vi "Dresden R2R Sputter 03.02.2018 IY24.vi"() -> ()   [LabVIEW 2009] (continued)
          }
          frame #9 {
            n6832 = flat-sequence {
              frame #0 {
                n6833 = Wait (ms)(milliseconds to wait=i32? 100) -> ()  [unwired: 1 out]
              }
              frame #1 {
                n6834 = local write "DC_auto_voltage_mode"(i16? 0 ("DC_auto_voltage_mode")) -> ()
              }
            }
            n6835 = VISA Write(VISA resource name=w10558, write buffer=bytes[4], error in (no error)=w10557) -> (VISA resource name out=w10556, error out=w10555)  [unwired: 1 out]
          }
        }
      }
    }
  }
  n6836 = call <vilib>:"MB Serial Init.vi"("Timeout"=i32? 2000, "Mode"=w750, "Parity"=w752, "Baud Rate"=i32? 9600, "VISA resource name"="Moxa I/O Ch 4") -> ("error out"=w756:errorcluster, "VISA resource name out"=w755:refnum<visa-resource-name>)  [unwired: 2 in, 3 out]
  n6837 = call <vilib>:"MB Serial Init.vi"("Timeout"=i32? 2000, "Mode"=w766, "Parity"=w764, "Baud Rate"=i32? 9600, "VISA resource name"="Moxa I/O Ch 3") -> ("error out"=w760:errorcluster, "VISA resource name out"=w761:refnum<visa-resource-name>)  [unwired: 2 in, 3 out]
  n6838 = while {
    tunnel: w814 -> [w10986]
    tunnel: w813 -> [w10985]
    shift-right: [w10811] -> _
    shift-left: _ -> [w10810]
    tunnel: [w10734] -> w809
    tunnel: [w10733] -> w733
    stop <- i16? 0 stop-if-true
    w10624 = bytes[2]
    w10586 = bytes[2]
    # "guc kaynagı ACK gelınceye kadar bekler."
    # "ACK karsılıgı 06(hex) dır."
    n6839 = Tick Count (ms)() -> (millisecond timer value=w10811)
    n6840 = Or(x="set rf", y="RF set auto") -> (x .or. y?=w10570)
    n6841 = Or(x="RF on", y="RF_auto_on") -> (x .or. y?=w10581)
    n6842 = Or(x="oto tuner", y="RF_auto_tuner") -> (x .or. y?=w10562)
    n6843 = Or(x="RF off", y="RF_auto_off") -> (x .or. y?=w10579)
    n6844 = Or(x="RF host", y="RF_host_auto") -> (x .or. y?=w10576)
    n6845 = Subtract(x=w10811, y=w10810) -> (x-y=→"x-y")
    n6846 = Or(x="Ramp Up time", y="Ramp Up time_auto") -> (x .or. y?=w10574)
    n6847 = Boolean To (0,1)(Boolean=w10576) -> (0, 1=w10960)
    n6848 = Boolean To (0,1)(Boolean=w10579) -> (0, 1=w10961)
    n6849 = Boolean To (0,1)(Boolean=w10581) -> (0, 1=w10967)
    n6850 = Boolean To (0,1)(Boolean=w10570) -> (0, 1=w10966)
    n6851 = Boolean To (0,1)(Boolean=w10562) -> (0, 1=w10965)
    n6852 = Boolean To (0,1)(Boolean="initialize") -> (0, 1=w10963)
    n6853 = Boolean To (0,1)(Boolean="Load") -> (0, 1=w10688)
    n6854 = Boolean To (0,1)(Boolean="Forward") -> (0, 1=w10685)
    n6855 = Boolean To (0,1)(Boolean="External") -> (0, 1=w10691)
    n6856 = Boolean To (0,1)(Boolean="Pulsing_off") -> (0, 1=w10698)
    n6857 = Boolean To (0,1)(Boolean="internal") -> (0, 1=w10699)
    n6858 = Boolean To (0,1)(Boolean="external") -> (0, 1=w10701)
    n6859 = Boolean To (0,1)(Boolean="set duty") -> (0, 1=w10714)
    n6860 = Boolean To (0,1)(Boolean=w10574) -> (0, 1=w10673)
    n6861 = Boolean To (0,1)(Boolean="manuel tuner") -> (0, 1=w10964)
    n6862 = Boolean To (0,1)(Boolean="set cap pos") -> (0, 1=w10962)
    n6863 = Boolean To (0,1)(Boolean="set seri cap pos 2") -> (0, 1=w10959)
    n6864 = Boolean To (0,1)(Boolean="set frequency") -> (0, 1=w10710)
    n6865 = Multiply(x=w10960, y=i16? 1) -> (x*y=w10683)
    n6866 = Multiply(x=w10961, y=i16? 3) -> (x*y=w10980)
    n6867 = Multiply(x=w10967, y=i16? 4) -> (x*y=w10981)
    n6868 = Multiply(x=w10966, y=i16? 5) -> (x*y=w10978)
    n6869 = Multiply(x=w10965, y=i16? 6) -> (x*y=w10976)
    n6870 = Multiply(x=w10963, y=i16? 8) -> (x*y=w10972)
    n6871 = Or(x="Ramp down time", y="Ramp Down time_auto") -> (x .or. y?=w10569)
    n6872 = Boolean To (0,1)(Boolean=w10569) -> (0, 1=w10671)
    n6873 = Multiply(x=w10964, y=i16? 7) -> (x*y=w10974)
    n6874 = Multiply(x=w10962, y=i16? 9) -> (x*y=w10970)
    n6875 = Multiply(x=w10688, y=i16? 2) -> (x*y=w10708)
    n6876 = Multiply(x=w10959, y=i16? 10) -> (x*y=w10968)
    n6877 = Multiply(x=w10685, y=i16? 11) -> (x*y=w10707)
    n6878 = Multiply(x=w10691, y=i16? 12) -> (x*y=w10706)
    n6879 = Multiply(x=w10698, y=i16? 13) -> (x*y=w10703)
    n6880 = Multiply(x=w10699, y=i16? 14) -> (x*y=w10704)
    n6881 = Multiply(x=w10701, y=i16? 15) -> (x*y=w10705)
    n6882 = Multiply(x=w10710, y=i16? 16) -> (x*y=w10712)
    n6883 = Multiply(x=w10714, y=i16? 17) -> (x*y=w10716)
    n6884 = Multiply(x=w10673, y=i16? 18) -> (x*y=w10670)
    n6885 = Multiply(x=w10671, y=i16? 19) -> (x*y=w10669)
    n6886 = String To Byte Array(string=w10586) -> (unsigned byte array=w10668)
    n6887 = for {
      tunnel: w10668 -> [w11022] mode=indexing
      shift-right: [w11020] -> w10666
      shift-left: data[5B] -> [w11021]
      n6888 = Exclusive Or(1:w11021, 2:w11022) -> (0:w11020)
    }
    n6889 = Compound Arithmetic op=ADD(w10708, w10707, w10706, w10703, w10704, w10705, w10712, w10716) -> (w10684)
    n6890 = Build Array(w10666) -> (w10665)
    n6891 = Compound Arithmetic op=ADD(w10683, w10980, w10981, w10978, w10976, w10974, w10972, w10970, w10968, w10684, w10670, w10669) -> (w10956)
    n6892 = Byte Array To String(unsigned byte array=w10665) -> (string=w10664)
    n6893 = Not Equal To 0?(x=w10956) -> (x != 0?=w10955)
    n6894 = case shown="3" w10956 {
      tunnel: [w11133 w11138 w11141 w11155 w11161 w11168 w11192 w11207 w11223 w11243 w11268 w11284 w11298 w11312 w11326 w11340 w11354 w11382 w11402 w11427] -> w10958
      tunnel: [w11132 w11137 w11140 w11156 w11162 w11169 w11191 w11206 w11224 w11242 w11267 w11283 w11297 w11311 w11325 w11339 w11353 w11381 w11401 w11426] -> w10957
      tunnel: w10986 -> [w11133 w11136 w11143 w11158 w11164 w11171 w11194 w11209 w11222 w11245 w11270 w11286 w11300 w11314 w11328 w11342 w11356 w11384 w11404 w11429]
      tunnel: w10985 -> [w11132 w11135 w11142 w11157 w11163 w11170 w11193 w11208 w11221 w11244 w11269 w11285 w11299 w11313 w11327 w11341 w11355 w11383 w11403 w11428]
      frame #0 {
      }
      frame #1 {
        # "Host kontrol"
        n6895 = local write "RF_host_auto"(i16? 0 ("RF_host_auto")) -> ()
        n6896 = VISA Write(VISA resource name=w11136, write buffer=bytes[4], error in (no error)=w11135) -> (VISA resource name out=w11138, error out=w11137)  [unwired: 1 out]
      }
      frame #2 {
        w11150 = bytes[3]
        n6897 = String To Byte Array(string=w11150) -> (unsigned byte array=w11144)
        n6898 = for {
          tunnel: w11144 -> [w11153] mode=indexing
          shift-right: [w11151] -> w11146
          shift-left: data[5B] -> [w11152]
          n6899 = Exclusive Or(1:w11152, 2:w11153) -> (0:w11151)
        }
        n6900 = Build Array(w11146) -> (w11148)
        n6901 = Byte Array To String(unsigned byte array=w11148) -> (string=w11147)
        n6902 = Concatenate Strings(w11150, w11147) -> (w11149)
        n6903 = VISA Write(VISA resource name=w11143, write buffer=w11149, error in (no error)=w11142) -> (VISA resource name out=w11141, error out=w11140)  [unwired: 1 out]
      }
      frame #3 {
        # "RF OFF"
        n6904 = local write "RF_auto_off"(i16? 0 ("RF_auto_off")) -> ()
        n6905 = VISA Write(VISA resource name=w11158, write buffer=bytes[3], error in (no error)=w11157) -> (VISA resource name out=w11155, error out=w11156)  [unwired: 1 out]
      }
      frame #4 {
        # "RF ON"
        n6906 = local write "RF_auto_on"(i16? 0 ("RF_auto_on")) -> ()
        n6907 = VISA Write(VISA resource name=w11164, write buffer=bytes[3], error in (no error)=w11163) -> (VISA resource name out=w11161, error out=w11162)  [unwired: 1 out]
      }
      frame #5 {
        n6908 = local write "RF set auto"(i16? 0 ("RF set auto")) -> ()
        n6909 = Quotient & Remainder(x="RF_forward_power_1", y=dbl? 256.0) -> (x-y*floor(x/y)=w11178, floor(x/y)=w11174)
        n6910 = Build Array(w11178) -> (w11177)
        n6911 = Build Array(w11174) -> (w11175)
        n6912 = Byte Array To String(unsigned byte array=w11177) -> (string=w11176)
        n6913 = Byte Array To String(unsigned byte array=w11175) -> (string=w11173)
        n6914 = Concatenate Strings(bytes[2], w11176, w11173) -> (w11180)
        n6915 = String To Byte Array(string=w11180) -> (unsigned byte array=w11186)
        n6916 = for {
          tunnel: w11186 -> [w11189] mode=indexing
          shift-right: [w11187] -> w11184
          shift-left: data[5B] -> [w11188]
          n6917 = Exclusive Or(1:w11188, 2:w11189) -> (0:w11187)
        }
        n6918 = Build Array(w11184) -> (w11183)
        n6919 = Byte Array To String(unsigned byte array=w11183) -> (string=w11181)
        n6920 = Concatenate Strings(w11180, w11181) -> (w11172)
        n6921 = VISA Write(VISA resource name=w11171, write buffer=w11172, error in (no error)=w11170) -> (VISA resource name out=w11168, error out=w11169)  [unwired: 1 out]
      }
      frame #6 {
        n6922 = Concatenate Strings(bytes[3]) -> (w11196)
        n6923 = local write "RF_auto_tuner"(i16? 0 ("RF_auto_tuner")) -> ()
        n6924 = String To Byte Array(string=w11196) -> (unsigned byte array=w11202)
        n6925 = for {
          tunnel: w11202 -> [w11205] mode=indexing
          shift-right: [w11203] -> w11200
          shift-left: data[5B] -> [w11204]
          n6926 = Exclusive Or(1:w11204, 2:w11205) -> (0:w11203)
        }
        n6927 = Build Array(w11200) -> (w11199)
        n6928 = Byte Array To String(unsigned byte array=w11199) -> (string=w11197)
        n6929 = Concatenate Strings(w11196, w11197) -> (w11195)
        n6930 = VISA Write(VISA resource name=w11194, write buffer=w11195, error in (no error)=w11193) -> (VISA resource name out=w11192, error out=w11191)  [unwired: 1 out]
      }
      frame #7 {
        n6931 = Concatenate Strings(bytes[3]) -> (w11211)
        n6932 = String To Byte Array(string=w11211) -> (unsigned byte array=w11217)
        n6933 = for {
          tunnel: w11217 -> [w11220] mode=indexing
          shift-right: [w11218] -> w11215
          shift-left: data[5B] -> [w11219]
          n6934 = Exclusive Or(1:w11219, 2:w11220) -> (0:w11218)
        }
        n6935 = Build Array(w11215) -> (w11214)
        n6936 = Byte Array To String(unsigned byte array=w11214) -> (string=w11212)
        n6937 = Concatenate Strings(w11211, w11212) -> (w11210)
        n6938 = VISA Write(VISA resource name=w11209, write buffer=w11210, error in (no error)=w11208) -> (VISA resource name out=w11207, error out=w11206)  [unwired: 1 out]
      }
      frame #8 {
        w11228 = bytes[2]
        n6939 = String To Byte Array(string=w11228) -> (unsigned byte array=w11231)
        n6940 = for {
          tunnel: w11231 -> [w11234] mode=indexing
          shift-right: [w11232] -> w11229
          shift-left: data[5B] -> [w11233]
          n6941 = Exclusive Or(1:w11233, 2:w11234) -> (0:w11232)
        }
        n6942 = Build Array(w11229) -> (w11226)
        n6943 = Byte Array To String(unsigned byte array=w11226) -> (string=w11227)
        n6944 = Concatenate Strings(w11228, w11227) -> (w11225)
        n6945 = VISA Write(VISA resource name=w11222, write buffer=w11225, error in (no error)=w11221) -> (VISA resource name out=w11223, error out=w11224)  [unwired: 1 out]
      }
      frame #9 {
        n6946 = Multiply(x="Set CL Position:", y=dbl? 10.0) -> (x*y=w11237)
        n6947 = To Unsigned Long Integer(number=w11237) -> (unsigned 32bit integer=w11236)
        n6948 = Quotient & Remainder(x=w11236, y=i32? 256) -> (x-y*floor(x/y)=w11241, floor(x/y)=w11240)
        n6949 = Build Array(w11241, w11240) -> (w11248)
        n6950 = Byte Array To String(unsigned byte array=w11248) -> (string=w11247)
        n6951 = Concatenate Strings("\np", w11247) -> (w11249)
        n6952 = String To Byte Array(string=w11249) -> (unsigned byte array=w11255)
        n6953 = for {
          tunnel: w11255 -> [w11258] mode=indexing
          shift-right: [w11256] -> w11253
          shift-left: data[5B] -> [w11257]
          n6954 = Exclusive Or(1:w11257, 2:w11258) -> (0:w11256)
        }
        n6955 = Build Array(w11253) -> (w11252)
        n6956 = Byte Array To String(unsigned byte array=w11252) -> (string=w11250)
        n6957 = Concatenate Strings(w11249, w11250) -> (w11246)
        n6958 = VISA Write(VISA resource name=w11245, write buffer=w11246, error in (no error)=w11244) -> (VISA resource name out=w11243, error out=w11242)  [unwired: 1 out]
      }
      frame #10 {
        n6959 = Multiply(x="Set CT Position:", y=dbl? 10.0) -> (x*y=w11259)
        n6960 = To Unsigned Long Integer(number=w11259) -> (unsigned 32bit integer=w11260)
        n6961 = Quotient & Remainder(x=w11260, y=i32? 256) -> (x-y*floor(x/y)=w11265, floor(x/y)=w11264)
        n6962 = Build Array(w11265, w11264) -> (w11262)
        n6963 = Byte Array To String(unsigned byte array=w11262) -> (string=w11272)
        n6964 = Concatenate Strings("\nz", w11272) -> (w11273)
        n6965 = String To Byte Array(string=w11273) -> (unsigned byte array=w11279)
        n6966 = for {
          tunnel: w11279 -> [w11282] mode=indexing
          shift-right: [w11280] -> w11277
          shift-left: data[5B] -> [w11281]
          n6967 = Exclusive Or(1:w11281, 2:w11282) -> (0:w11280)
        }
        n6968 = Build Array(w11277) -> (w11276)
        n6969 = Byte Array To String(unsigned byte array=w11276) -> (string=w11274)
        n6970 = Concatenate Strings(w11273, w11274) -> (w11271)
        n6971 = VISA Write(VISA resource name=w11270, write buffer=w11271, error in (no error)=w11269) -> (VISA resource name out=w11268, error out=w11267)  [unwired: 1 out]
      }
      frame #11 {
        w11290 = bytes[3]
        n6972 = String To Byte Array(string=w11290) -> (unsigned byte array=w11287)
        n6973 = for {
          tunnel: w11287 -> [w11296] mode=indexing
          shift-right: [w11294] -> w11289
          shift-left: data[5B] -> [w11295]
          n6974 = Exclusive Or(1:w11295, 2:w11296) -> (0:w11294)
        }
        n6975 = Build Array(w11289) -> (w11291)
        n6976 = Byte Array To String(unsigned byte array=w11291) -> (string=w11292)
        n6977 = Concatenate Strings(w11290, w11292) -> (w11293)
        n6978 = VISA Write(VISA resource name=w11286, write buffer=w11293, error in (no error)=w11285) -> (VISA resource name out=w11284, error out=w11283)  [unwired: 1 out]
      }
      frame #12 {
        w11305 = bytes[3]
        n6979 = String To Byte Array(string=w11305) -> (unsigned byte array=w11301)
        n6980 = for {
          tunnel: w11301 -> [w11310] mode=indexing
          shift-right: [w11308] -> w11303
          shift-left: data[5B] -> [w11309]
          n6981 = Exclusive Or(1:w11309, 2:w11310) -> (0:w11308)
        }
        n6982 = Build Array(w11303) -> (w11304)
        n6983 = Byte Array To String(unsigned byte array=w11304) -> (string=w11306)
        n6984 = Concatenate Strings(w11305, w11306) -> (w11307)
        n6985 = VISA Write(VISA resource name=w11300, write buffer=w11307, error in (no error)=w11299) -> (VISA resource name out=w11298, error out=w11297)  [unwired: 1 out]
      }
      frame #13 {
        w11319 = bytes[3]
        n6986 = String To Byte Array(string=w11319) -> (unsigned byte array=w11315)
        n6987 = for {
          tunnel: w11315 -> [w11324] mode=indexing
          shift-right: [w11322] -> w11317
          shift-left: data[5B] -> [w11323]
          n6988 = Exclusive Or(1:w11323, 2:w11324) -> (0:w11322)
        }
        n6989 = Build Array(w11317) -> (w11318)
        n6990 = Byte Array To String(unsigned byte array=w11318) -> (string=w11320)
        n6991 = Concatenate Strings(w11319, w11320) -> (w11321)
        n6992 = VISA Write(VISA resource name=w11314, write buffer=w11321, error in (no error)=w11313) -> (VISA resource name out=w11312, error out=w11311)  [unwired: 1 out]
      }
      frame #14 {
        w11335 = bytes[3]
        n6993 = String To Byte Array(string=w11335) -> (unsigned byte array=w11329)
        n6994 = for {
          tunnel: w11329 -> [w11338] mode=indexing
          shift-right: [w11336] -> w11331
          shift-left: data[5B] -> [w11337]
          n6995 = Exclusive Or(1:w11337, 2:w11338) -> (0:w11336)
        }
        n6996 = Build Array(w11331) -> (w11332)
        n6997 = Byte Array To String(unsigned byte array=w11332) -> (string=w11333)
        n6998 = Concatenate Strings(w11335, w11333) -> (w11334)
        n6999 = VISA Write(VISA resource name=w11328, write buffer=w11334, error in (no error)=w11327) -> (VISA resource name out=w11326, error out=w11325)  [unwired: 1 out]
      }
      frame #15 {
        w11347 = bytes[3]
        n7000 = String To Byte Array(string=w11347) -> (unsigned byte array=w11343)
        n7001 = for {
          tunnel: w11343 -> [w11352] mode=indexing
          shift-right: [w11350] -> w11345
          shift-left: data[5B] -> [w11351]
          n7002 = Exclusive Or(1:w11351, 2:w11352) -> (0:w11350)
        }
        n7003 = Build Array(w11345) -> (w11346)
        n7004 = Byte Array To String(unsigned byte array=w11346) -> (string=w11348)
        n7005 = Concatenate Strings(w11347, w11348) -> (w11349)
        n7006 = VISA Write(VISA resource name=w11342, write buffer=w11349, error in (no error)=w11341) -> (VISA resource name out=w11340, error out=w11339)  [unwired: 1 out]
      }
      frame #16 {
        w11369 = dbl? 256.0 ("y")
        n7007 = Quotient & Remainder(x="Frequency :", y=w11369) -> (x-y*floor(x/y)=w11364, floor(x/y)=w11368)
        n7008 = Build Array(w11364) -> (w11365)
        n7009 = Quotient & Remainder(x=w11368, y=w11369) -> (x-y*floor(x/y)=w11370, floor(x/y)=w11374)
        n7010 = Byte Array To String(unsigned byte array=w11365) -> (string=w11372)
        n7011 = Build Array(w11370) -> (w11371)
        n7012 = Build Array(w11374) -> (w11366)
        n7013 = Byte Array To String(unsigned byte array=w11371) -> (string=w11375)
        n7014 = Byte Array To String(unsigned byte array=w11366) -> (string=w11376)
        n7015 = Concatenate Strings(bytes[2], w11372, w11375, w11376, bytes[1] ("string")) -> (w11363)
        n7016 = String To Byte Array(string=w11363) -> (unsigned byte array=w11357)
        n7017 = for {
          tunnel: w11357 -> [w11380] mode=indexing
          shift-right: [w11378] -> w11359
          shift-left: data[5B] -> [w11379]
          n7018 = Exclusive Or(1:w11379, 2:w11380) -> (0:w11378)
        }
        n7019 = Build Array(w11359) -> (w11360)
        n7020 = Byte Array To String(unsigned byte array=w11360) -> (string=w11362)
        n7021 = Concatenate Strings(w11363, w11362) -> (w11377)
        n7022 = VISA Write(VISA resource name=w11356, write buffer=w11377, error in (no error)=w11355) -> (VISA resource name out=w11354, error out=w11353)  [unwired: 1 out]
      }
      frame #17 {
        n7023 = Build Array("Duty Cycle :") -> (w11394)
        n7024 = Byte Array To String(unsigned byte array=w11394) -> (string=w11395)
        n7025 = Concatenate Strings("\n`", w11395, bytes[1] ("string")) -> (w11391)
        n7026 = String To Byte Array(string=w11391) -> (unsigned byte array=w11385)
        n7027 = for {
          tunnel: w11385 -> [w11399] mode=indexing
          shift-right: [w11397] -> w11387
          shift-left: data[5B] -> [w11398]
          n7028 = Exclusive Or(1:w11398, 2:w11399) -> (0:w11397)
        }
        n7029 = Build Array(w11387) -> (w11388)
        n7030 = Byte Array To String(unsigned byte array=w11388) -> (string=w11390)
        n7031 = Concatenate Strings(w11391, w11390) -> (w11396)
        n7032 = VISA Write(VISA resource name=w11384, write buffer=w11396, error in (no error)=w11383) -> (VISA resource name out=w11382, error out=w11381)  [unwired: 1 out]
      }
      frame #18 {
        n7033 = Multiply(x="Ramp up Time:", y=dbl? 10.0) -> (x*y=w11408)
        n7034 = To Unsigned Long Integer(number=w11408) -> (unsigned 32bit integer=w11407)
        n7035 = local write "Ramp Up time_auto"(i16? 0 ("Ramp Up time_auto")) -> ()
        n7036 = Quotient & Remainder(x=w11407, y=i32? 256) -> (x-y*floor(x/y)=w11411, floor(x/y)=w11410)
        n7037 = Build Array(w11411, w11410) -> (w11406)
        n7038 = Byte Array To String(unsigned byte array=w11406) -> (string=w11414)
        n7039 = Concatenate Strings(bytes[2], w11414) -> (w11415)
        n7040 = String To Byte Array(string=w11415) -> (unsigned byte array=w11421)
        n7041 = for {
          tunnel: w11421 -> [w11424] mode=indexing
          shift-right: [w11422] -> w11419
          shift-left: data[5B] -> [w11423]
          n7042 = Exclusive Or(1:w11423, 2:w11424) -> (0:w11422)
        }
        n7043 = Build Array(w11419) -> (w11418)
        n7044 = Byte Array To String(unsigned byte array=w11418) -> (string=w11416)
        n7045 = Concatenate Strings(w11415, w11416) -> (w11413)
        n7046 = VISA Write(VISA resource name=w11404, write buffer=w11413, error in (no error)=w11403) -> (VISA resource name out=w11402, error out=w11401)  [unwired: 1 out]
      }
      frame #19 {
        n7047 = Multiply(x="Ramp Down Time :", y=dbl? 10.0) -> (x*y=w11433)
        n7048 = To Unsigned Long Integer(number=w11433) -> (unsigned 32bit integer=w11432)
        n7049 = local write "Ramp Down time_auto"(i16? 0 ("Ramp Down time_auto")) -> ()
        n7050 = Quotient & Remainder(x=w11432, y=i32? 256) -> (x-y*floor(x/y)=w11436, floor(x/y)=w11435)
        n7051 = Build Array(w11436, w11435) -> (w11431)
        n7052 = Byte Array To String(unsigned byte array=w11431) -> (string=w11439)
        n7053 = Concatenate Strings("\n ", w11439) -> (w11440)
        n7054 = String To Byte Array(string=w11440) -> (unsigned byte array=w11446)
        n7055 = for {
          tunnel: w11446 -> [w11449] mode=indexing
          shift-right: [w11447] -> w11444
          shift-left: data[5B] -> [w11448]
          n7056 = Exclusive Or(1:w11448, 2:w11449) -> (0:w11447)
        }
        n7057 = Build Array(w11444) -> (w11443)
        n7058 = Byte Array To String(unsigned byte array=w11443) -> (string=w11441)
        n7059 = Concatenate Strings(w11440, w11441) -> (w11438)
        n7060 = VISA Write(VISA resource name=w11429, write buffer=w11438, error in (no error)=w11428) -> (VISA resource name out=w11427, error out=w11426)  [unwired: 1 out]
      }
    }
    n7061 = Concatenate Strings(w10586, w10664) -> (w10657)
    n7062 = case shown="True" w10955 {
      tunnel: w10958 -> [w11116 w11126]
      tunnel: w10957 -> [w11115 w11125]
      tunnel: [w11116 w11128] -> w10945
      tunnel: [w11115 w11122] -> w10944
      frame #0 {
      }
      frame #1 {
        n7063 = stacked-sequence {
          tunnel: [w11131] -> w11124
          tunnel: w11126 -> [w11131]
          tunnel: [w11130] -> w11123
          tunnel: w11125 -> [w11130]
          frame #0 {
            n7064 = Wait Until Next ms Multiple(millisecond multiple=i32? 40) -> ()  [unwired: 1 out]
          }
        }
        n7065 = property class="Instr"(reference=w11124, error in=w11123) -> (reference out=w11121, error out=w11120, "Serial Settings:Number of Bytes at Serial Port"=w11119)
        n7066 = VISA Read(VISA resource name=w11121, byte count=w11119, error in (no error)=w11120) -> (VISA resource name out=w11118, error out=w11117)  [unwired: 2 out]
        n7067 = VISA Write(VISA resource name=w11118, write buffer=bytes[1], error in (no error)=w11117) -> (VISA resource name out=w11128, error out=w11122)  [unwired: 1 out]
      }
    }
    n7068 = VISA Write(VISA resource name=w10945, write buffer=bytes[3], error in (no error)=w10944) -> (VISA resource name out=w10950, error out=w10949)  [unwired: 1 out]
    n7069 = stacked-sequence {
      tunnel: [w11114] -> w10947
      tunnel: w10950 -> [w11114]
      tunnel: [w11113] -> w10946
      tunnel: w10949 -> [w11113]
      frame #0 {
        n7070 = Wait Until Next ms Multiple(millisecond multiple=i32? 40) -> ()  [unwired: 1 out]
      }
    }
    n7071 = property class="Instr"(reference=w10947, error in=w10946) -> (reference out=w10951, error out=w10953, "Serial Settings:Number of Bytes at Serial Port"=w10952)
    n7072 = VISA Read(VISA resource name=w10951, byte count=w10952, error in (no error)=w10953) -> (VISA resource name out=w10595, read buffer=w10943, error out=w10594)  [unwired: 1 out]
    n7073 = Match Pattern(string=w10943, regular expression="¦") -> (after substring=w10591)  [unwired: 4 out]
    n7074 = String Length(string=w10591) -> (length=w10942)
    n7075 = String Subset(string=w10591, length (rest)=i32? 2 ("length (rest)")) -> (substring=w10940)  [unwired: 1 out]
    n7076 = Not Equal To 0?(x=w10942) -> (x != 0?=w10588)
    n7077 = String To Byte Array(string=w10940) -> (unsigned byte array=w10938)
    n7078 = case shown="True" w10588 {
      tunnel: [w10989 w10993] -> w10593
      tunnel: [w10988 w10992] -> w10592
      tunnel: w10595 -> [w10989 w10991]
      tunnel: w10594 -> [w10988 w10990]
      frame #0 {
      }
      frame #1 {
        n7079 = VISA Write(VISA resource name=w10991, write buffer=bytes[1], error in (no error)=w10990) -> (VISA resource name out=w10993, error out=w10992)  [unwired: 1 out]
      }
    }
    n7080 = Index Array(array=w10938, index=i32? 1) -> (element=w10934)
    n7081 = Index Array(array=w10938, index=data[5B]) -> (element=w10932)
    n7082 = To Unsigned Long Integer(number=w10934) -> (unsigned 32bit integer=w10936)
    n7083 = To Unsigned Long Integer(number=w10932) -> (unsigned 32bit integer=w10931)
    n7084 = Multiply(x=i32? 256, y=w10936) -> (x*y=w10933)
    n7085 = Add(x=w10933, y=w10931) -> (x+y=w10682)
    n7086 = case shown="True" w10588 {
      tunnel: w10682 -> [_ w11041]
      frame #0 {
      }
      frame #1 {
        "Reflected Power" <- w11041
      }
    }
    n7087 = VISA Write(VISA resource name=w10593, write buffer=w10657, error in (no error)=w10592) -> (VISA resource name out=w10661, error out=w10660)  [unwired: 1 out]
    n7088 = stacked-sequence {
      tunnel: [w11019] -> w10659
      tunnel: w10661 -> [w11019]
      tunnel: [w11018] -> w10658
      tunnel: w10660 -> [w11018]
      frame #0 {
        n7089 = Wait Until Next ms Multiple(millisecond multiple=i32? 40) -> ()  [unwired: 1 out]
      }
    }
    n7090 = property class="Instr"(reference=w10659, error in=w10658) -> (reference out=w10662, error out=w10663, "Serial Settings:Number of Bytes at Serial Port"=w10587)
    n7091 = VISA Read(VISA resource name=w10662, byte count=w10587, error in (no error)=w10663) -> (VISA resource name out=w10644, read buffer=w10654, error out=w10643)  [unwired: 1 out]
    n7092 = Match Pattern(string=w10654, regular expression="¢") -> (after substring=w10652)  [unwired: 4 out]
    n7093 = String Length(string=w10652) -> (length=w10656)
    n7094 = String Subset(string=w10652, length (rest)=i32? 1 ("length (rest)")) -> (substring=w10650)  [unwired: 1 out]
    n7095 = String To Byte Array(string=w10650) -> (unsigned byte array=w10649)
    n7096 = Not Equal To 0?(x=w10656) -> (x != 0?=w10655)
    n7097 = Index Array(array=w10649, index=data[5B]) -> (element=w10647)
    n7098 = String To Byte Array(string=w10624) -> (unsigned byte array=w10629)
    n7099 = Number To Boolean Array(number=w10647) -> (Boolean array=w10646)
    n7100 = case shown="True" w10655 {
      tunnel: [w11011 w11015] -> w10597
      tunnel: [w11010 w11014] -> w10596
      tunnel: w10644 -> [w11011 w11013]
      tunnel: w10643 -> [w11010 w11012]
      frame #0 {
      }
      frame #1 {
        n7101 = VISA Write(VISA resource name=w11013, write buffer=bytes[1], error in (no error)=w11012) -> (VISA resource name out=w11015, error out=w11014)  [unwired: 1 out]
      }
    }
    n7102 = for {
      tunnel: w10629 -> [w10999] mode=indexing
      shift-right: [w10997] -> w10627
      shift-left: data[5B] -> [w10998]
      n7103 = Exclusive Or(1:w10998, 2:w10999) -> (0:w10997)
    }
    n7104 = Index Array(array=w10646, index=i32? 6) -> (element=→"RF 1 On")
    n7105 = Build Array(w10627) -> (w10626)
    n7106 = Byte Array To String(unsigned byte array=w10626) -> (string=w10625)
    n7107 = Concatenate Strings(w10624, w10625) -> (w10623)
    n7108 = VISA Write(VISA resource name=w10597, write buffer=w10623, error in (no error)=w10596) -> (VISA resource name out=w10639, error out=w10638)  [unwired: 1 out]
    n7109 = stacked-sequence {
      tunnel: [w11009] -> w10635
      tunnel: w10639 -> [w11009]
      tunnel: [w11008] -> w10634
      tunnel: w10638 -> [w11008]
      frame #0 {
        n7110 = Wait Until Next ms Multiple(millisecond multiple=i32? 40) -> ()  [unwired: 1 out]
      }
    }
    n7111 = property class="Instr"(reference=w10635, error in=w10634) -> (reference out=w10641, error out=w10640, "Serial Settings:Number of Bytes at Serial Port"=w10599)
    n7112 = VISA Read(VISA resource name=w10641, byte count=w10599, error in (no error)=w10640) -> (VISA resource name out=w10633, read buffer=w10636, error out=w10632)  [unwired: 1 out]
    n7113 = Match Pattern(string=w10636, regular expression="—") -> (after substring=w10630)  [unwired: 4 out]
    n7114 = String Length(string=w10630) -> (length=w10631)
    n7115 = String To Byte Array(string=w10630) -> (unsigned byte array=w10602)
    n7116 = Not Equal To 0?(x=w10631) -> (x != 0?=w10598)
    n7117 = Index Array(array=w10602, index=i32? 1) -> (element=w10618)
    n7118 = Index Array(array=w10602, index=data[5B]) -> (element=w10615)
    n7119 = Index Array(array=w10602, index=i32? 3) -> (element=w10613)
    n7120 = Index Array(array=w10602, index=i32? 2) -> (element=w10612)
    n7121 = To Unsigned Long Integer(number=w10618) -> (unsigned 32bit integer=w10617)
    n7122 = To Unsigned Long Integer(number=w10615) -> (unsigned 32bit integer=w10614)
    n7123 = To Unsigned Long Integer(number=w10613) -> (unsigned 32bit integer=w10610)
    n7124 = To Unsigned Long Integer(number=w10612) -> (unsigned 32bit integer=w10611)
    n7125 = case shown="True" w10598 {
      tunnel: w10633 -> [w11001 w11005]
      tunnel: w10632 -> [w11000 w11004]
      tunnel: [w11001 w11003] -> w10590
      tunnel: [w11000 w11002] -> w10589
      frame #0 {
      }
      frame #1 {
        n7126 = VISA Write(VISA resource name=w11005, write buffer=bytes[1], error in (no error)=w11004) -> (VISA resource name out=w11003, error out=w11002)  [unwired: 1 out]
      }
    }
    n7127 = local read "Forward Power"() -> (w10585)
    n7128 = local read "Reflected Power"() -> (w10584)
    n7129 = Multiply(x=w10617, y=i32? 256) -> (x*y=w10620)
    n7130 = Multiply(x=i32? 256, y=w10610) -> (x*y=w10608)
    n7131 = Add(x=w10620, y=w10614) -> (x+y=w10603)
    n7132 = Add(x=w10608, y=w10611) -> (x+y=w10604)
    n7133 = Subtract(x=w10585, y=w10584) -> (x-y=→"RF Net Power :")
    n7134 = Divide(x=w10603, y=i32? 10) -> (x/y=w10601)
    n7135 = Divide(x=w10604, y=i32? 10) -> (x/y=w10600)
    n7136 = case shown="True" w10598 {
      tunnel: w10601 -> [_ w10996]
      tunnel: w10600 -> [_ w10995]
      frame #0 {
      }
      frame #1 {
        "Ramp Up Left Time:" <- w10996
        "Ramp Down Left Time:" <- w10995
      }
    }
    n7137 = VISA Write(VISA resource name=w10590, write buffer=bytes[3], error in (no error)=w10589) -> (VISA resource name out=w10912, error out=w10910)  [unwired: 1 out]
    n7138 = stacked-sequence {
      tunnel: [w11110] -> w10913
      tunnel: w10912 -> [w11110]
      tunnel: [w11109] -> w10911
      tunnel: w10910 -> [w11109]
      frame #0 {
        n7139 = Wait Until Next ms Multiple(millisecond multiple=i32? 40) -> ()  [unwired: 1 out]
      }
    }
    n7140 = property class="Instr"(reference=w10913, error in=w10911) -> (reference out=w10928, error out=w10927, "Serial Settings:Number of Bytes at Serial Port"=w10929)
    n7141 = VISA Read(VISA resource name=w10928, byte count=w10929, error in (no error)=w10927) -> (VISA resource name out=w10909, read buffer=w10914, error out=w10908)  [unwired: 1 out]
    n7142 = Match Pattern(string=w10914, regular expression="¥") -> (after substring=w10906)  [unwired: 4 out]
    n7143 = String Length(string=w10906) -> (length=w10907)
    n7144 = String Subset(string=w10906, length (rest)=i32? 2 ("length (rest)")) -> (substring=w10924)  [unwired: 1 out]
    n7145 = Not Equal To 0?(x=w10907) -> (x != 0?=w10681)
    n7146 = String To Byte Array(string=w10924) -> (unsigned byte array=w10922)
    n7147 = case shown="True" w10681 {
      tunnel: w10909 -> [w11103 w11107]
      tunnel: w10908 -> [w11102 w11106]
      tunnel: [w11103 w11105] -> w10884
      tunnel: [w11102 w11104] -> w10883
      frame #0 {
      }
      frame #1 {
        n7148 = VISA Write(VISA resource name=w11107, write buffer=bytes[1], error in (no error)=w11106) -> (VISA resource name out=w11105, error out=w11104)  [unwired: 1 out]
      }
    }
    n7149 = Index Array(array=w10922, index=i32? 1) -> (element=w10919)
    n7150 = Index Array(array=w10922, index=data[5B]) -> (element=w10916)
    n7151 = To Unsigned Long Integer(number=w10919) -> (unsigned 32bit integer=w10918)
    n7152 = To Unsigned Long Integer(number=w10916) -> (unsigned 32bit integer=w10915)
    n7153 = Multiply(x=i32? 256, y=w10918) -> (x*y=w10917)
    n7154 = Add(x=w10917, y=w10915) -> (x+y=w10730)
    n7155 = case shown="True" w10681 {
      tunnel: w10730 -> [_ w11040]
      frame #0 {
      }
      frame #1 {
        "Forward Power" <- w11040
      }
    }
    n7156 = VISA Write(VISA resource name=w10884, write buffer=bytes[3], error in (no error)=w10883) -> (VISA resource name out=w10889, error out=w10888)  [unwired: 1 out]
    n7157 = stacked-sequence {
      tunnel: [w11101] -> w10887
      tunnel: w10889 -> [w11101]
      tunnel: [w11100] -> w10886
      tunnel: w10888 -> [w11100]
      frame #0 {
        n7158 = Wait Until Next ms Multiple(millisecond multiple=i32? 40) -> ()  [unwired: 1 out]
      }
    }
    n7159 = property class="Instr"(reference=w10887, error in=w10886) -> (reference out=w10905, error out=w10903, "Serial Settings:Number of Bytes at Serial Port"=w10904)
    n7160 = VISA Read(VISA resource name=w10905, byte count=w10904, error in (no error)=w10903) -> (VISA resource name out=w10882, read buffer=w10902, error out=w10881)  [unwired: 1 out]
    n7161 = Match Pattern(string=w10902, regular expression="¨") -> (after substring=w10880)  [unwired: 4 out]
    n7162 = String Length(string=w10880) -> (length=w10879)
    n7163 = String Subset(string=w10880, length (rest)=i32? 2 ("length (rest)")) -> (substring=w10899)  [unwired: 1 out]
    n7164 = Not Equal To 0?(x=w10879) -> (x != 0?=w10680)
    n7165 = String To Byte Array(string=w10899) -> (unsigned byte array=w10897)
    n7166 = case shown="True" w10680 {
      tunnel: w10882 -> [w11093 w11097]
      tunnel: w10881 -> [w11092 w11096]
      tunnel: [w11093 w11095] -> w10843
      tunnel: [w11092 w11094] -> w10836
      frame #0 {
      }
      frame #1 {
        n7167 = VISA Write(VISA resource name=w11097, write buffer=bytes[1], error in (no error)=w11096) -> (VISA resource name out=w11095, error out=w11094)  [unwired: 1 out]
      }
    }
    n7168 = Index Array(array=w10897, index=i32? 1) -> (element=w10892)
    n7169 = Index Array(array=w10897, index=data[5B]) -> (element=w10893)
    n7170 = To Unsigned Long Integer(number=w10892) -> (unsigned 32bit integer=w10895)
    n7171 = To Unsigned Long Integer(number=w10893) -> (unsigned 32bit integer=w10890)
    n7172 = Multiply(x=i32? 256, y=w10895) -> (x*y=w10891)
    n7173 = Add(x=w10891, y=w10890) -> (x+y=w10729)
    n7174 = case shown="True" w10680 {
      tunnel: w10729 -> [_ w11039]
      frame #0 {
      }
      frame #1 {
        "DC Bias:" <- w11039
      }
    }
    n7175 = VISA Write(VISA resource name=w10843, write buffer=bytes[3], error in (no error)=w10836) -> (VISA resource name out=w10875, error out=w10874)  [unwired: 1 out]
    n7176 = stacked-sequence {
      tunnel: [w11091] -> w10848
      tunnel: w10875 -> [w11091]
      tunnel: [w11090] -> w10847
      tunnel: w10874 -> [w11090]
      frame #0 {
        n7177 = Wait Until Next ms Multiple(millisecond multiple=i32? 40) -> ()  [unwired: 1 out]
      }
    }
    n7178 = property class="Instr"(reference=w10848, error in=w10847) -> (reference out=w10877, error out=w10876, "Serial Settings:Number of Bytes at Serial Port"=w10878)
    n7179 = VISA Read(VISA resource name=w10877, byte count=w10878, error in (no error)=w10876) -> (VISA resource name out=w10842, read buffer=w10849, error out=w10841)  [unwired: 1 out]
    n7180 = Match Pattern(string=w10849, regular expression="¯") -> (after substring=w10839)  [unwired: 4 out]
    n7181 = String Length(string=w10839) -> (length=w10840)
    n7182 = String Subset(string=w10839, length (rest)=i32? 2 ("length (rest)")) -> (substring=w10866)  [unwired: 1 out]
    n7183 = String Subset(string=w10839, offset (0)=i32? 2, length (rest)=i32? 2 ("length (rest)")) -> (substring=w10861)
    n7184 = Not Equal To 0?(x=w10840) -> (x != 0?=w10679)
    n7185 = String To Byte Array(string=w10866) -> (unsigned byte array=w10869)
    n7186 = String To Byte Array(string=w10861) -> (unsigned byte array=w10863)
    n7187 = case shown="True" w10679 {
      tunnel: [w11083 w11087] -> w10817
      tunnel: [w11082 w11086] -> w10816
      tunnel: w10842 -> [w11083 w11085]
      tunnel: w10841 -> [w11082 w11084]
      frame #0 {
      }
      frame #1 {
        n7188 = VISA Write(VISA resource name=w11085, write buffer=bytes[1], error in (no error)=w11084) -> (VISA resource name out=w11087, error out=w11086)  [unwired: 1 out]
      }
    }
    n7189 = Index Array(array=w10869, index=i32? 1) -> (element=w10860)
    n7190 = Index Array(array=w10869, index=data[5B]) -> (element=w10857)
    n7191 = Index Array(array=w10863, index=i32? 1) -> (element=w10855)
    n7192 = Index Array(array=w10863, index=data[5B]) -> (element=w10854)
    n7193 = To Unsigned Long Integer(number=w10860) -> (unsigned 32bit integer=w10859)
    n7194 = To Unsigned Long Integer(number=w10857) -> (unsigned 32bit integer=w10856)
    n7195 = To Unsigned Long Integer(number=w10855) -> (unsigned 32bit integer=w10852)
    n7196 = To Unsigned Long Integer(number=w10854) -> (unsigned 32bit integer=w10853)
    n7197 = Multiply(x=w10859, y=i32? 256) -> (x*y=w10867)
    n7198 = Multiply(x=i32? 256, y=w10852) -> (x*y=w10850)
    n7199 = Add(x=w10867, y=w10856) -> (x+y=w10837)
    n7200 = Add(x=w10850, y=w10853) -> (x+y=w10838)
    n7201 = case shown="True" w10679 {
      tunnel: i32? 10 ("y") -> [_ w11038]
      tunnel: i32? 10 ("y") -> [_ w11037]
      tunnel: w10838 -> [_ w11036]
      tunnel: w10837 -> [_ w11035]
      frame #0 {
      }
      frame #1 {
        n7202 = Divide(x=w11035, y=w11038) -> (x/y=→"CL Position:")
        n7203 = Divide(x=w11036, y=w11037) -> (x/y=→"CT Position:")
      }
    }
    n7204 = VISA Write(VISA resource name=w10817, write buffer=bytes[3], error in (no error)=w10816) -> (VISA resource name out=w10832, error out=w10831)  [unwired: 1 out]
    n7205 = stacked-sequence {
      tunnel: [w11081] -> w10819
      tunnel: w10832 -> [w11081]
      tunnel: [w11080] -> w10818
      tunnel: w10831 -> [w11080]
      frame #0 {
        n7206 = Wait Until Next ms Multiple(millisecond multiple=i32? 40) -> ()  [unwired: 1 out]
      }
    }
    n7207 = property class="Instr"(reference=w10819, error in=w10818) -> (reference out=w10834, error out=w10833, "Serial Settings:Number of Bytes at Serial Port"=w10835)
    n7208 = VISA Read(VISA resource name=w10834, byte count=w10835, error in (no error)=w10833) -> (VISA resource name out=w10815, read buffer=w10820, error out=w10814)  [unwired: 1 out]
    n7209 = Match Pattern(string=w10820, regular expression=bytes[3]) -> (after substring=w10812)  [unwired: 4 out]
    n7210 = String Length(string=w10812) -> (length=w10813)
    n7211 = String Subset(string=w10812, length (rest)=i32? 1 ("length (rest)")) -> (substring=w10821)  [unwired: 1 out]
    n7212 = Not Equal To 0?(x=w10813) -> (x != 0?=w10678)
    n7213 = Match True/False String(2:data[5B] ("false string"), 3:bytes[1] ("true string"), 4:w10821) -> (0:w10728)  [unwired: 1 out]
    n7214 = Match True/False String(2:data[5B] ("false string"), 3:bytes[1] ("true string"), 4:w10821) -> (0:w10727)  [unwired: 1 out]
    n7215 = Match True/False String(2:data[5B] ("false string"), 3:bytes[1] ("true string"), 4:w10821) -> (0:w10726)  [unwired: 1 out]
    n7216 = case shown="True" w10678 {
      tunnel: [w11073 w11077] -> w10791
      tunnel: [w11072 w11074] -> w10790
      tunnel: w10815 -> [w11073 w11076]
      tunnel: w10814 -> [w11072 w11075]
      frame #0 {
      }
      frame #1 {
        n7217 = VISA Write(VISA resource name=w11076, write buffer=bytes[1], error in (no error)=w11075) -> (VISA resource name out=w11077, error out=w11074)  [unwired: 1 out]
      }
    }
    n7218 = case shown="True" w10678 {
      tunnel: w10728 -> [_ w11032]
      tunnel: w10727 -> [_ w11031]
      tunnel: w10726 -> [_ w11030]
      frame #0 {
      }
      frame #1 {
        "FORWARD   REGULATION" <- w11032
        "LOAD  REGULATION" <- w11030
        "DC BIAS REGULATION" <- w11031
      }
    }
    n7219 = VISA Write(VISA resource name=w10791, write buffer=bytes[3], error in (no error)=w10790) -> (VISA resource name out=w10805, error out=w10804)  [unwired: 1 out]
    n7220 = stacked-sequence {
      tunnel: [w11071] -> w10793
      tunnel: w10805 -> [w11071]
      tunnel: [w11070] -> w10792
      tunnel: w10804 -> [w11070]
      frame #0 {
        n7221 = Wait Until Next ms Multiple(millisecond multiple=i32? 40) -> ()  [unwired: 1 out]
      }
    }
    n7222 = property class="Instr"(reference=w10793, error in=w10792) -> (reference out=w10807, error out=w10806, "Serial Settings:Number of Bytes at Serial Port"=w10808)
    n7223 = VISA Read(VISA resource name=w10807, byte count=w10808, error in (no error)=w10806) -> (VISA resource name out=w10789, read buffer=w10794, error out=w10788)  [unwired: 1 out]
    n7224 = Match Pattern(string=w10794, regular expression="±") -> (after substring=w10786)  [unwired: 4 out]
    n7225 = String Subset(string=w10786) -> (substring=w10795)  [unwired: 2 out]
    n7226 = String Length(string=w10786) -> (length=w10787)
    n7227 = Not Equal To 0?(x=w10787) -> (x != 0?=w10677)
    n7228 = Match True/False String(2:data[5B] ("false string"), 3:bytes[1] ("true string"), 4:w10795) -> (0:w10725)  [unwired: 1 out]
    n7229 = Match True/False String(2:data[5B] ("false string"), 3:bytes[1] ("true string"), 4:w10795) -> (0:w10724)  [unwired: 1 out]
    n7230 = Match True/False String(2:data[5B] ("false string"), 3:bytes[1] ("true string"), 4:w10795) -> (0:w10723)  [unwired: 1 out]
    n7231 = case shown="True" w10677 {
      tunnel: [w11063 w11065] -> w10773
      tunnel: [w11062 w11064] -> w10772
      tunnel: w10789 -> [w11063 w11067]
      tunnel: w10788 -> [w11062 w11066]
      frame #0 {
      }
      frame #1 {
        n7232 = VISA Write(VISA resource name=w11067, write buffer=bytes[1], error in (no error)=w11066) -> (VISA resource name out=w11065, error out=w11064)  [unwired: 1 out]
      }
    }
    n7233 = case shown="True" w10677 {
      tunnel: w10725 -> [_ w11029]
      tunnel: w10724 -> [_ w11028]
      tunnel: w10723 -> [_ w11026]
      frame #0 {
      }
      frame #1 {
        n7234 = Not(x=w11028) -> (.not. x?=w11027)
        n7235 = And(x=w11027, y=w11026) -> (x .and. y?=→"Pulsing ON/OFF :")
        "INTERNAL PULSING" <- w11026
        "PULSING OFF" <- w11028
        "EXTERNAL PULSING" <- w11029
      }
    }
    n7236 = VISA Write(VISA resource name=w10773, write buffer=bytes[3], error in (no error)=w10772) -> (VISA resource name out=w10782, error out=w10781)  [unwired: 1 out]
    n7237 = stacked-sequence {
      tunnel: [w11061] -> w10775
      tunnel: w10782 -> [w11061]
      tunnel: [w11060] -> w10774
      tunnel: w10781 -> [w11060]
      frame #0 {
        n7238 = Wait Until Next ms Multiple(millisecond multiple=i32? 40) -> ()  [unwired: 1 out]
      }
    }
    n7239 = property class="Instr"(reference=w10775, error in=w10774) -> (reference out=w10784, error out=w10783, "Serial Settings:Number of Bytes at Serial Port"=w10785)
    n7240 = VISA Read(VISA resource name=w10784, byte count=w10785, error in (no error)=w10783) -> (VISA resource name out=w10771, read buffer=w10776, error out=w10770)  [unwired: 1 out]
    n7241 = Match Pattern(string=w10776, regular expression="Ä") -> (after substring=w10768)  [unwired: 4 out]
    n7242 = String To Byte Array(string=w10768) -> (unsigned byte array=w10778)
    n7243 = String Length(string=w10768) -> (length=w10676)
    n7244 = Not Equal To 0?(x=w10676) -> (x != 0?=w10769)
    n7245 = Index Array(array=w10778, index=data[5B]) -> (element=w10722)
    n7246 = case shown="1" w10676 {
      tunnel: w10722 -> [_ w11024]
      frame #0 {
      }
      frame #1 {
        "duty cycle" <- w11024
      }
    }
    n7247 = case shown="True" w10769 {
      tunnel: [w11053 w11055] -> w10738
      tunnel: [w11052 w11054] -> w10737
      tunnel: w10771 -> [w11053 w11057]
      tunnel: w10770 -> [w11052 w11056]
      frame #0 {
      }
      frame #1 {
        n7248 = VISA Write(VISA resource name=w11057, write buffer=bytes[1], error in (no error)=w11056) -> (VISA resource name out=w11055, error out=w11054)  [unwired: 1 out]